vi "CRYO_MASTER_FULL_dev.vi"() -> ()   [LabVIEW 2017] (continued)
  out "P (1K pot)":dbl=100068.27348256127 format="%_4e"
  out "P (3He pot)":dbl=99910.45562672244 format="%_4e"
  out "P (shield return)":dbl=99525.03881922836 format="%_4e"
  out "P (3He IN)":dbl=99868.7240011457 format="%_4e"
  out "P (4K reservoir)":dbl=99802.94678056413 format="%_4e"
  out "P (insulation)":dbl=0.0001474505418094343 format="%_4e"
  in  "1Kpot pump exhaust flow":string="F_5"
  out "F_5":dbl=37.619829557129414 format="%_4f"
  in  "3He incoming flow into HEX7":string="F_4"
  out "F_4":dbl=-7.249983269540847 format="%_4f"
  out "F_3":dbl=-0.052681534547558584 format="%_4f"
  in  "4He return flow from HEX7":string="F_3"
  out "F_2":dbl=-0.13159086515246687 format="%_4f"
  in  "Shield flow":string="F_2"
  out "P_SldRTN":dbl=99525.03881922836 format="%_4e"
  in  "3He pot pressure":string="P_3Hepot"
  out "P_3Hepot":dbl=99910.45562672244 format="%_4e"
  in  "Shield return press.":string="P_SldRTN"
  out "F_1":dbl=3.609913543945148 format="%_4f"
  in  "3He pump exhaust flow":string="F_1"
  out "P_Dewar":dbl=100437.10701708468 format="%_4e"
  in  "Dewar pressure":string="P_Dewar"
  out "P_1Kpot":dbl=100068.27348256127 format="%_4e"
  in  "1Kpot pressure":string="P_1Kpot"
  out "P_3HeIN":dbl=99868.7240011457 format="%_4e"
  in  "3He inlet pressure":string="P_3HeIN"
  in  "4K reservoir pressure":string="P_4Kres"
  out "P_4Kres":dbl=99802.94678056413 format="%_4e"
  out "P_ins":dbl=0.0001474505418094343 format="%_4e"
  in  "Insulation vacuum":string="P_ins"
  out "T3He7-1/6-2 (3He pot) 2":dbl=8.3718 format="%_4f"
  out "T3He7-1/7-2 (HEX1)":dbl=8.4614 format="%_4f"
  out "T3He6-1/6-2 (3He pot) 2":dbl=8.4997 format="%_4f"
  out "T3He6-1/6-2 (HEX1)":dbl=8.4934 format="%_4f"
  out "T1K3-1/3-2 (1K pot) 2":dbl=4.1883 format="%_4f"
  out "T1K3-1/3-2 (1K pot)":dbl=4.1814 format="%_4f"
  out "T4He1 (4K reservoir )":dbl=4.447 format="%_4f"
  out "Temperature 1":dbl=19.065
  in  "SensorLocation 1":T14(ring)=enum."TTH2"
  out "TIP7":dbl format="%_4g"
  out "T3He6-2":dbl=8.4997 format="%_4g"
  out "T3He7-2":dbl=8.3718 format="%_4g"
  out "T3He6-1":dbl=8.4934 format="%_4g"
  out "T3He4":dbl=9.675 format="%_4g"
  out "T3He7-1":dbl=8.4614 format="%_4g"
  out "T3He8":dbl=8.8291 format="%_4g"
  out "T3He5":dbl=4.3215 format="%_4g"
  out "T1K3-2":dbl=4.1883 format="%_4g"
  out "T1K3-1":dbl=4.1814 format="%_4g"
  out "TIP6":dbl=18.257 format="%_4g"
  out "T3He9":dbl=10.682 format="%_4g"
  out "T1K5":dbl=4.692 format="%_4g"
  out "T1K4":dbl=4.458 format="%_4g"
  out "T1K2":dbl=4.216 format="%_4g"
  out "TIP5":dbl=17.346 format="%_4g"
  out "TIP4":dbl=11.053 format="%_4g"
  out "TIP3":dbl=39.061 format="%_4g"
  out "TIP2":dbl=88.205 format="%_4g"
  out "TIP1":dbl=246.21 format="%_4g"
  out "T1K6":dbl=250.44 format="%_4g"
  out "T4He10":dbl=208.38 format="%_4g"
  out "T4He8":dbl=166.06 format="%_4g"
  out "T4He7":dbl=115.68 format="%_4g"
  out "T3He1-3":dbl=277.53 format="%_4g"
  out "T3He1-2":dbl=279.51 format="%_4g"
  out "T4He9":dbl=97.885 format="%_4g"
  out "T4He6":dbl=25.122 format="%_4g"
  out "T4He5":dbl=25.726 format="%_4g"
  out "T4He4":dbl=30.925 format="%_4g"
  out "T4He2-2":dbl=35.069 format="%_4g"
  out "T4He2-1":dbl=34.286 format="%_4g"
  out "T4He3-4":dbl=285.55 format="%_4g"
  out "T4He3-3":dbl=285.5 format="%_4g"
  out "T4He3-2":dbl=287.85 format="%_4g"
  out "T4He3-1":dbl=287.74 format="%_4g"
  out "T3He1-4":dbl=276.97 format="%_4g"
  out "T3He3":dbl=17.248 format="%_4g"
  out "T3He2-2":dbl=34.793 format="%_4g"
  out "T3He2-1":dbl=46.023 format="%_4g"
  out "T1K1":dbl=10.801 format="%_4g"
  out "T4He1":dbl=4.447 format="%_4g"
  out "TTH1":dbl=19.184 format="%_4g"
  out "TTH2":dbl=19.065 format="%_4g"
  out "TTH4":dbl=112.53 format="%_4g"
  out "TTH3":dbl=106.31 format="%_4g"
  out "T3He1-1":dbl=279.64 format="%_4g"
  out "T3He10":dbl=250.64 format="%_4g"
  out "F2 (shield flow)":dbl=-0.13159086515246687 format="%_4f"
  out "DP_HEX4":dbl=-42.27649010016066 format="%_4e"
  in  "4K reservoir level":string="L3"
  out "L3":dbl=0.05537433565456876 format="%_4f"
  out "RUN Identifier 6":string="20201120_195613_RUNII" caption="RUN Identifier"
  in  "HEX7 out pressure":string="P_HEX7OUT"
  in  "STOP CHF":bool
  in  "CHF Graph Comment":string="CHF_Warmup"
  in  "REFRESH GRAPH":bool
  in  "RECORD GRAPH":bool
  out "Graph CHF log 2":T4(graph) caption="XY Graph"
  out "ƒ¢T_array":dbl[](array[numeric])=[-0.0029999999999998916, -0.0031999999999998696, -0.0031999999999998696, -0.0031999999999998696, -0.0030999999999998806, -0.0030999999999998806, -0.0031999999999998696, -0.0033999999999998476, -0.0030999999999998806, -0.0032999999999998586, -0.0028999999999999027, -0.0032999999999998586, -0.0030999999999998806, -0.0032999999999998586, -0.0030999999999998806, -0.0030999999999998806, -0.0030999999999998806, -0.0031999999999998696, -0.0031999999999998696, -0.0029999999999998916, -0.0028999999999999027, -0.0029999999999998916, -0.0032000000000000917, -0.0030000000000001137, -0.0031000000000001027, -0.0027000000000001467, -0.0029000000000001247, -0.0029000000000001247, -0.0031000000000001027, -0.0025999999999999357, -0.0027999999999999137, -0.0025999999999999357, -0.0027999999999999137, -0.0024999999999999467, -0.0028999999999999027, -0.0023999999999999577, -0.0023000000000001908, -0.0023999999999999577, -0.0026999999999999247, -0.0024999999999999467, -0.0023999999999999577, -0.0024999999999999467, -0.0023999999999999577, -0.0025000000000001688, -0.0020000000000000018, -0.0022999999999999687, -0.002100000000000213, -0.0020000000000000018, -0.0020999999999999908, -0.0016000000000000458, -0.0019000000000000128, -0.0014000000000000679, -0.0017000000000000348, -0.0013000000000000789, -0.0013999999999998458, -0.0011999999999998678, -0.0016000000000000458, -0.0017000000000000348, -0.0009000000000001229, -0.0012000000000000899, -0.0008000000000001339, -0.001000000000000112, -0.0012000000000000899, -0.0010999999999998789, -0.0009000000000001229, -0.0010999999999998789, -0.0019000000000000128, -0.0016000000000000458, -0.0008999999999999009, -0.0004999999999999449, -0.0009000000000001229, -0.0011999999999998678, -0.0006999999999997009, -0.00010000000000021103, -0.0010999999999996568, -0.001100000000000101, -0.0008999999999996788, 0.00010000000000021103, -0.000700000000000145, -0.00039999999999995595, 0.0, -0.00010000000000021103, 0.00019999999999997797, -0.0009999999999998899, 0.00019999999999997797, -0.000700000000000145, 0.000600000000000378, -0.0006999999999997009, 0.0015999999999998238, 0.0015999999999998238, 0.010199999999999765, 0.00140000000000029, 0.0038999999999997925, -0.007899999999999796, 0.0028999999999999027, -0.004100000000000215, 0.006000000000000227, 0.0034000000000000696, 0.0, -0.0026000000000001577, 0.0013000000000000789, -0.013700000000000045, 0.0015000000000000568, 0.0038000000000000256, 0.000300000000000189, -0.0034000000000000696, -0.00019999999999997797, -0.0009000000000001229, -0.0049000000000001265, -0.0017000000000000348, 0.0020999999999999908, 0.000700000000000145, 0.0024999999999999467, 0.0011999999999998678, 0.0043999999999999595, 0.001200000000000312, -0.0009999999999998899, -0.00039999999999995595, 0.0027999999999996916, 0.0020999999999999908, 0.0028000000000001357, 0.0028000000000001357, 0.0038000000000000256, 0.006200000000000205, 0.001100000000000101, 0.0040000000000000036, 0.0024999999999999467, 0.005300000000000082, 0.0027000000000003688, 0.0032000000000000917, 0.0046000000000003816, 0.0045000000000001705, 0.00550000000000006, 0.0038999999999997925, 0.0045999999999999375, 0.0032999999999998586, 0.0039000000000002366, 0.0028000000000001357, 0.0019999999999997797, 0.0040000000000000036, 0.0013999999999998458, 0.006600000000000161, 0.0015999999999998238, 0.0045000000000001705, 0.02400000000000002, 0.012199999999999989, 0.0049000000000001265, 0.014599999999999724, 0.0043999999999999595, 0.013900000000000023, 0.007899999999999796, 0.014200000000000212, 0.08460000000000001, 0.0038000000000000256, 0.014199999999999768, 0.029699999999999616, 0.051200000000000134, 0.09330000000000016, 0.28469999999999995, 1.3064, 0.7519, 0.9085000000000001, 3.6559, 3.1087999999999996, 3.1484000000000005, 4.376900000000001, 4.8179, 5.180999999999999, 5.6812000000000005, 6.102599999999999, 6.5953, 6.675800000000001, 7.3666, 7.8156, 8.344, 8.904599999999999, 8.9488, 9.2997, 9.7916, 10.0504, 10.446399999999999, 10.966099999999999, 11.3154, 11.6655, 12.011, 12.4506, 12.629000000000001, 12.9298, 13.34, 13.658900000000001, 14.0009, 14.365399999999998, 14.6644, 14.959400000000002, 15.242600000000001, 15.613299999999999, 15.9224, 16.2284, 16.4516, 16.7094]
  out "Graph CHF":cluster{dbl[], dbl[]}(graph)={[-0.0029999999999998916, -0.0031999999999998696, -0.0031999999999998696, -0.0031999999999998696, -0.0030999999999998806, -0.0030999999999998806, -0.0031999999999998696, -0.0033999999999998476, -0.0030999999999998806, -0.0032999999999998586, -0.0028999999999999027, -0.0032999999999998586, -0.0030999999999998806, -0.0032999999999998586, -0.0030999999999998806, -0.0030999999999998806, -0.0030999999999998806, -0.0031999999999998696, -0.0031999999999998696, -0.0029999999999998916, -0.0028999999999999027, -0.0029999999999998916, -0.0032000000000000917, -0.0030000000000001137, -0.0031000000000001027, -0.0027000000000001467, -0.0029000000000001247, -0.0029000000000001247, -0.0031000000000001027, -0.0025999999999999357, -0.0027999999999999137, -0.0025999999999999357, -0.0027999999999999137, -0.0024999999999999467, -0.0028999999999999027, -0.0023999999999999577, -0.0023000000000001908, -0.0023999999999999577, -0.0026999999999999247, -0.0024999999999999467, -0.0023999999999999577, -0.0024999999999999467, -0.0023999999999999577, -0.0025000000000001688, -0.0020000000000000018, -0.0022999999999999687, -0.002100000000000213, -0.0020000000000000018, -0.0020999999999999908, -0.0016000000000000458, -0.0019000000000000128, -0.0014000000000000679, -0.0017000000000000348, -0.0013000000000000789, -0.0013999999999998458, -0.0011999999999998678, -0.0016000000000000458, -0.0017000000000000348, -0.0009000000000001229, -0.0012000000000000899, -0.0008000000000001339, -0.001000000000000112, -0.0012000000000000899, -0.0010999999999998789, -0.0009000000000001229, -0.0010999999999998789, -0.0019000000000000128, -0.0016000000000000458, -0.0008999999999999009, -0.0004999999999999449, -0.0009000000000001229, -0.0011999999999998678, -0.0006999999999997009, -0.00010000000000021103, -0.0010999999999996568, -0.001100000000000101, -0.0008999999999996788, 0.00010000000000021103, -0.000700000000000145, -0.00039999999999995595, 0.0, -0.00010000000000021103, 0.00019999999999997797, -0.0009999999999998899, 0.00019999999999997797, -0.000700000000000145, 0.000600000000000378, -0.0006999999999997009, 0.0015999999999998238, 0.0015999999999998238, 0.010199999999999765, 0.00140000000000029, 0.0038999999999997925, -0.007899999999999796, 0.0028999999999999027, -0.004100000000000215, 0.006000000000000227, 0.0034000000000000696, 0.0, -0.0026000000000001577, 0.0013000000000000789, -0.013700000000000045, 0.0015000000000000568, 0.0038000000000000256, 0.000300000000000189, -0.0034000000000000696, -0.00019999999999997797, -0.0009000000000001229, -0.0049000000000001265, -0.0017000000000000348, 0.0020999999999999908, 0.000700000000000145, 0.0024999999999999467, 0.0011999999999998678, 0.0043999999999999595, 0.001200000000000312, -0.0009999999999998899, -0.00039999999999995595, 0.0027999999999996916, 0.0020999999999999908, 0.0028000000000001357, 0.0028000000000001357, 0.0038000000000000256, 0.006200000000000205, 0.001100000000000101, 0.0040000000000000036, 0.0024999999999999467, 0.005300000000000082, 0.0027000000000003688, 0.0032000000000000917, 0.0046000000000003816, 0.0045000000000001705, 0.00550000000000006, 0.0038999999999997925, 0.0045999999999999375, 0.0032999999999998586, 0.0039000000000002366, 0.0028000000000001357, 0.0019999999999997797, 0.0040000000000000036, 0.0013999999999998458, 0.006600000000000161, 0.0015999999999998238, 0.0045000000000001705, 0.02400000000000002, 0.012199999999999989, 0.0049000000000001265, 0.014599999999999724, 0.0043999999999999595, 0.013900000000000023, 0.007899999999999796, 0.014200000000000212, 0.08460000000000001, 0.0038000000000000256, 0.014199999999999768, 0.029699999999999616, 0.051200000000000134, 0.09330000000000016, 0.28469999999999995, 1.3064, 0.7519, 0.9085000000000001, 3.6559, 3.1087999999999996, 3.1484000000000005, 4.376900000000001, 4.8179, 5.180999999999999, 5.6812000000000005, 6.102599999999999, 6.5953, 6.675800000000001, 7.3666, 7.8156, 8.344, 8.904599999999999, 8.9488, 9.2997, 9.7916, 10.0504, 10.446399999999999, 10.966099999999999, 11.3154, 11.6655, 12.011, 12.4506, 12.629000000000001, 12.9298, 13.34, 13.658900000000001, 14.0009, 14.365399999999998, 14.6644, 14.959400000000002, 15.242600000000001, 15.613299999999999, 15.9224, 16.2284, 16.4516, 16.7094], [0.00177179408, 0.0047188563824, 0.009062122761600002, 0.014841429971200002, 0.022050593188799993, 0.030674497986, 0.0406770254784, 0.0520756828592, 0.0652426793424, 0.07951245148399999, 0.095196614256, 0.11212304208000001, 0.13146225656, 0.15140636999200002, 0.172767285228, 0.19523839632000003, 0.22089373680000002, 0.24639792231999996, 0.27309037243199996, 0.300834606864, 0.333309042144, 0.364200416856, 0.396376777992, 0.428969786608, 0.46852352470399994, 0.5048892, 0.5415947771520001, 0.5780588070400001, 0.62555439864, 0.6656076272399999, 0.7053064507, 0.7438503797200001, 0.8028658319759999, 0.84516135816, 0.8855220791599998, 0.9243742466799998, 0.9987769028, 1.040549527104, 1.07657183264, 1.1053520089920001, 1.2023590229040002, 1.3125317079600003, 1.355469355336, 1.4108726480399998, 1.4642265462839996, 1.5508259575799999, 1.609969226688, 1.6681944120439995, 1.7212315581999997, 1.8197203732960001, 1.8816147001599999, 1.939246332968, 1.993681569632, 2.110421822528, 2.1715208164760003, 2.2300658826359996, 2.33203464608, 2.4312324865440003, 2.520524222848, 2.56333261656, 2.661313337984, 2.7867724064, 2.8377456422800003, 2.963749773600001, 3.01323235824, 3.143606416840001, 3.1874947393199995, 3.3286276941600006, 3.3671324332799997, 3.4297475918799996, 3.4776642959999995, 3.48994194976, 3.7174310035199993, 3.7518448211999993, 3.756501273839999, 3.8155461344, 4.26509900712, 4.04162726208, 4.09879309824, 4.5867353948, 4.69579370944, 4.39389811152, 4.9172907186399994, 5.029857857199999, 5.14319635, 5.257784033319999, 5.373066988079999, 5.48922905748, 5.606999167360001, 5.7253151114400005, 5.8451341704, 5.9653806828, 6.087172249440001, 6.20936272008, 6.3330874655999985, 6.457355812319998, 6.5829079103599994, 6.709043396000002, 6.836579179000002, 6.9645565727999985, 7.093596729600001, 7.223932919599999, 7.354796004800001, 7.486911963999998, 7.6198231199999995, 7.7532066848, 7.887716202000003, 8.024043540800001, 8.126487840000001, 8.269554521199998, 8.4077936336, 8.5471331664, 8.6875860064, 8.8284394528, 8.971763136, 9.114345182800001, 9.257739612, 9.403949720000002, 9.549304752000001, 9.695266022, 9.841513750000003, 9.99153291, 10.140170450400001, 10.289093019200001, 10.4378083004, 10.594207987199999, 10.7454584848, 10.897314274, 11.0478970848, 11.210433023999999, 11.363073264000002, 11.514230988000001, 11.6672069304, 11.8363924328, 11.990053261999998, 12.141437804, 12.316577644799997, 12.469949637600003, 12.6221502, 12.768815616000001, 12.9613889756, 13.112679096, 13.260713388, 13.3955342568, 13.6139294592, 13.767960665600002, 13.903996679999999, 14.0298325128, 14.272124848799997, 14.408208115599999, 14.535468526799997, 14.625996168000002, 14.9276629944, 15.049154579999998, 15.132236211999997, 15.444088045600003, 15.570016308800001, 15.687675859999997, 15.778474975199998, 16.133452762, 16.2316771404, 16.278357173599996, 16.259788331199996, 16.7384176632, 16.723491475199996, 16.714044836000003, 16.528176336, 17.254680908799997, 18.0156484144, 16.952834118, 18.4038018464, 18.599578232000002, 18.794163826000002, 18.99096738, 19.1888872744, 19.3889457516, 19.588486306799997, 19.789104642, 19.9907612412, 20.1933504, 20.396427222400003, 20.600519206399998, 20.8041637608, 21.010700178, 21.216750239999996, 21.4245511792, 21.632564418399998, 21.8418047652, 22.051294878, 22.26281235, 22.47403692, 22.68618526, 22.899439349999998, 23.111589312, 23.325939447999996, 23.540653440000003, 23.7536142072, 23.968794931199998, 24.183715353199997, 24.407023065599997]}
  in  "V_lim_low (V)":dbl format="%_5f"
  in  "V_lim_up (V)":dbl=120.0 format="%_5f"
  out "V":dbl=37.9024
  out "I":dbl=0.643944
  out "Q":dbl=24.407023065599997
  out "T_low":dbl=2.1656
  out "CHF log file name":string="20201120_102906_RUNII_20201120_154856_CHFlog.csv"
  in  "Data T_low":T15={"Source"=enum."LSI336", "SourceLabel"="T3He6-1"}
  in  "Data T_high":T15={"Source"=enum."LSI336", "SourceLabel"="T3He7-2"}
  in  "RecordSettings":T16(array[cluster])=[{"Source"=enum."DMMs", "SourceLabel"="I_H1", "FileFormat"="%4.4e"}, {"Source"=enum."DMMs", "SourceLabel"="V_H1", "FileFormat"="%4.4f"}, {"Source"=enum."USB6210", "SourceLabel"="P_3Hepot", "FileFormat"="%4.4e"}, {"Source"=enum."USB6218AI", "SourceLabel"="F_1", "FileFormat"="%4.4f"}, {"Source"=enum."USB6218AI", "SourceLabel"="F_4", "FileFormat"="%4.4f"}, {"Source"=enum."USB6218AI", "SourceLabel"="F_5", "FileFormat"="%4.4f"}, {"Source"=enum."USB6210", "SourceLabel"="DP_HEX4", "FileFormat"="%4.4e"}, {"Source"=enum."LSI336", "SourceLabel"="T3He6-1", "FileFormat"="%4.4f"}, {"Source"=enum."LSI336", "SourceLabel"="T3He6-2", "FileFormat"="%4.4f"}, {"Source"=enum."LSI336", "SourceLabel"="T3He7-1", "FileFormat"="%4.4f"}, {"Source"=enum."LSI336", "SourceLabel"="T3He7-2", "FileFormat"="%4.4f"}, {"Source"=enum."LSI336", "SourceLabel"="T1K3-1", "FileFormat"="%4.4f"}, {"Source"=enum."LSI336", "SourceLabel"="T1K3-2", "FileFormat"="%4.4f"}]
  in  "Data V":T15={"Source"=enum."DMMs", "SourceLabel"="V_H1"}
  in  "Data I":T15={"Source"=enum."DMMs", "SourceLabel"="I_H1"}
  in  "START CHF":bool
  in  "CHF cycle interval (s) (>1s)":dbl=1.0 format="%_3f"
  in  "V_end (V)":dbl=100.0 format="%_4f"
  in  "V start (V)":dbl format="%_4f"
  in  "ƒ¢V / cycle (V)":dbl=0.5 format="%_4f"
  out "error out (Agilent)":errorcluster
  in  "VISA (Agilent 34402)":refnum<visa-resource-name>="USB0::0x0957::0x0407::MY44010230::INSTR"
  out "Agilent\nIntialized?":bool=TRUE
  in  "Initialize (Agilent)":bool
  in  "OUTPUT \nKenwood":bool
  in  "Kenwood set V (V)":dbl min=0.0 max=120.0 format="%_5f"
  out "Graph CHF log 1":T4(graph) caption="XY Graph"
  out "CHF Data Labels":string[](array[string])=["I_H1", "V_H1", "P_3Hepot", "F_1", "F_4", "F_5", "DP_HEX4", "T3He6-1", "T3He6-2", "T3He7-1", "T3He7-2", "T1K3-1", "T1K3-2"]
  out "CHF last data":dbl[](array[numeric])=[0.643944, 37.9024, 3745.6366507925286, 1.653619757825851, -6.92448226263659, 35.2098077546946, -11.781018947359195, 2.1656, 6.7476, 2.1606, 18.875, 1.9567, 1.9598]
  out "Error out (CHF rec)":errorcluster
  out "CHF measurement counter":i32
  out "T_high":dbl=18.875
  out "ƒ¢T":dbl=16.7094
  out "Q_array":dbl[](array[numeric])=[0.00177179408, 0.0047188563824, 0.009062122761600002, 0.014841429971200002, 0.022050593188799993, 0.030674497986, 0.0406770254784, 0.0520756828592, 0.0652426793424, 0.07951245148399999, 0.095196614256, 0.11212304208000001, 0.13146225656, 0.15140636999200002, 0.172767285228, 0.19523839632000003, 0.22089373680000002, 0.24639792231999996, 0.27309037243199996, 0.300834606864, 0.333309042144, 0.364200416856, 0.396376777992, 0.428969786608, 0.46852352470399994, 0.5048892, 0.5415947771520001, 0.5780588070400001, 0.62555439864, 0.6656076272399999, 0.7053064507, 0.7438503797200001, 0.8028658319759999, 0.84516135816, 0.8855220791599998, 0.9243742466799998, 0.9987769028, 1.040549527104, 1.07657183264, 1.1053520089920001, 1.2023590229040002, 1.3125317079600003, 1.355469355336, 1.4108726480399998, 1.4642265462839996, 1.5508259575799999, 1.609969226688, 1.6681944120439995, 1.7212315581999997, 1.8197203732960001, 1.8816147001599999, 1.939246332968, 1.993681569632, 2.110421822528, 2.1715208164760003, 2.2300658826359996, 2.33203464608, 2.4312324865440003, 2.520524222848, 2.56333261656, 2.661313337984, 2.7867724064, 2.8377456422800003, 2.963749773600001, 3.01323235824, 3.143606416840001, 3.1874947393199995, 3.3286276941600006, 3.3671324332799997, 3.4297475918799996, 3.4776642959999995, 3.48994194976, 3.7174310035199993, 3.7518448211999993, 3.756501273839999, 3.8155461344, 4.26509900712, 4.04162726208, 4.09879309824, 4.5867353948, 4.69579370944, 4.39389811152, 4.9172907186399994, 5.029857857199999, 5.14319635, 5.257784033319999, 5.373066988079999, 5.48922905748, 5.606999167360001, 5.7253151114400005, 5.8451341704, 5.9653806828, 6.087172249440001, 6.20936272008, 6.3330874655999985, 6.457355812319998, 6.5829079103599994, 6.709043396000002, 6.836579179000002, 6.9645565727999985, 7.093596729600001, 7.223932919599999, 7.354796004800001, 7.486911963999998, 7.6198231199999995, 7.7532066848, 7.887716202000003, 8.024043540800001, 8.126487840000001, 8.269554521199998, 8.4077936336, 8.5471331664, 8.6875860064, 8.8284394528, 8.971763136, 9.114345182800001, 9.257739612, 9.403949720000002, 9.549304752000001, 9.695266022, 9.841513750000003, 9.99153291, 10.140170450400001, 10.289093019200001, 10.4378083004, 10.594207987199999, 10.7454584848, 10.897314274, 11.0478970848, 11.210433023999999, 11.363073264000002, 11.514230988000001, 11.6672069304, 11.8363924328, 11.990053261999998, 12.141437804, 12.316577644799997, 12.469949637600003, 12.6221502, 12.768815616000001, 12.9613889756, 13.112679096, 13.260713388, 13.3955342568, 13.6139294592, 13.767960665600002, 13.903996679999999, 14.0298325128, 14.272124848799997, 14.408208115599999, 14.535468526799997, 14.625996168000002, 14.9276629944, 15.049154579999998, 15.132236211999997, 15.444088045600003, 15.570016308800001, 15.687675859999997, 15.778474975199998, 16.133452762, 16.2316771404, 16.278357173599996, 16.259788331199996, 16.7384176632, 16.723491475199996, 16.714044836000003, 16.528176336, 17.254680908799997, 18.0156484144, 16.952834118, 18.4038018464, 18.599578232000002, 18.794163826000002, 18.99096738, 19.1888872744, 19.3889457516, 19.588486306799997, 19.789104642, 19.9907612412, 20.1933504, 20.396427222400003, 20.600519206399998, 20.8041637608, 21.010700178, 21.216750239999996, 21.4245511792, 21.632564418399998, 21.8418047652, 22.051294878, 22.26281235, 22.47403692, 22.68618526, 22.899439349999998, 23.111589312, 23.325939447999996, 23.540653440000003, 23.7536142072, 23.968794931199998, 24.183715353199997, 24.407023065599997]
  out "CHF file name":string="20201120_102906_RUNII_CHF20201120_155319_CHF_Warmup.csv"
  out "Graph CHF log 3":T4(graph) caption="XY Graph"
  out "File Refnum (CHF)":refnum<file>
  out "Series 1":string[](array[string])=["P_ins", "P_4Kres", "P_3HeIN", "P_SldRTN", "P_3Hepot", "P_1Kpot", "P_Dewar(old)", "P_HEX7OUT", "P_IP"]
  out "Series 2":string[](array[string])=["DP_HEX4", "DP_HEX5", "L1", "L2-1", "L2-2", "L3"]
  out "Series 3":string[](array[string])=["F_1", "F_2", "F_3", "F_4", "F_5", "I_CV", "P_Dewar"]
  out "Series 4":string[](array[string])=["TTH3", "TTH4", "TTH1", "TTH2", "T4He1", "T1K1", "T3He2-1", "T3He2-2", "T4He3-1", "T4He3-2", "T4He3-3", "T4He3-4", "T4He2-1", "T4He2-2", "T4He4", "T1K2", "T1K4", "T1K5", "T3He4", "T1K3-1", "T1K3-2", "T3He5", "T3He8", "T3He6-1", "T3He6-2", "T3He7-1", "T3He7-2"]
  out "Plot errors":errorcluster
  out "LastMeasurementConfig (218)":T17(array[cluster])=[{"LSIName"="LSI218A", "Active?"=TRUE, "LastData"=[250.64, 279.64, 106.3, 112.52, 19.165, 19.038, 4.436, 10.775], "Labels"=["T3He10", "T3He1-1", "TTH3", "TTH4", "TTH1", "TTH2", "T4He1", "T1K1"]}, {"LSIName"="LSI218B", "Active?"=TRUE, "LastData"=[30.0, 0.0, 0.0, 0.0, 46.025, 34.792, 17.25, 276.96], "Labels"=["N.C.", "N.C.", "N.C.", "N.C.", "T3He2-1", "T3He2-2", "T3He3", "T3He1-4"]}, {"LSIName"="LSI218C", "Active?"=TRUE, "LastData"=[287.74, 287.84, 285.5, 285.55, 34.292, 35.074, 30.928, 25.728], "Labels"=["T4He3-1", "T4He3-2", "T4He3-3", "T4He3-4", "T4He2-1", "T4He2-2", "T4He4", "T4He5"]}, {"LSIName"="LSI218D", "Active?"=TRUE, "LastData"=[25.125, 97.886, 279.52, 277.53, 115.69, 166.07, 208.39, 250.44], "Labels"=["T4He6", "T4He9", "T3He1-2", "T3He1-3", "T4He7", "T4He8", "T4He10", "T1K6"]}, {"LSIName"="LSI218E", "Active?"=TRUE, "LastData"=[246.21, 0.0, 88.2, 688.49, 39.062, 11.046, 17.368, 688.58], "Labels"=["TIP1", "N.C.", "TIP2", "N.C.", "TIP3", "TIP4", "TIP5", "N.C."]}, {"LSIName"="LSI218F", "Active?"=TRUE, "LastData"=[4.194, 4.476, 4.691, 9.636, 10.639, 18.262, 0.433, 0.0], "Labels"=["T1K2", "T1K4", "T1K5", "T3He4", "T3He9", "TIP6", "N.C.", "N.C."]}]
  out "DataArrayConv (USB6210)":dbl[][](array[numeric])
  out "LastMeasurementConfig (336)":T17(array[cluster])=[{"LSIName"="LSi336X", "Active?"=TRUE, "LastData"=[4.182, 4.1886, 4.3213, 8.8312], "Labels"=["T1K3-1", "T1K3-2", "T3He5", "T3He8"]}, {"LSIName"="LSi336Y", "Active?"=TRUE, "LastData"=[8.4926, 8.5004, 8.4614, 8.3712], "Labels"=["T3He6-1", "T3He6-2", "T3He7-1", "T3He7-2"]}]
  out "DataArrayConv (USB6218)":dbl[][](array[numeric])
  out "TimeArray (USB6218)":timestamp[](array[timestamp])
  out "Data Array sizes (6210)":i32[](array[numeric])=[33552, 16]
  out "DataArraySize (6218)":i32[](array[numeric])=[33552, 8]
  out "TimeArray size (6218)":i32=33552
  out "TimeArray (LSI336)":timestamp[](array[timestamp])
  out "TimeArray Size (336)":i32=33552
  out "DataArray (336)":dbl[][](array[numeric])
  out "DataArray size (336)":i32[](array[numeric])=[33552, 8]
  out "LastData (LSI218)":dbl[](array[numeric])=[250.64, 279.64, 106.3, 112.52, 19.165, 19.038, 4.436, 10.775, 30.0, 0.0, 0.0, 0.0, 46.025, 34.792, 17.25, 276.96, 287.74, 287.84, 285.5, 285.55, 34.292, 35.074, 30.928, 25.728, 25.125, 97.886, 279.52, 277.53, 115.69, 166.07, 208.39, 250.44, 246.21, 0.0, 88.2, 688.49, 39.062, 11.046, 17.368, 688.58, 4.194, 4.476, 4.691, 9.636, 10.639, 18.262, 0.433, 0.0]
  out "TempSensorsLocations":T18(array[ring])=[enum."T3He10", enum."T3He1-1", enum."TTH3", enum."TTH4", enum."TTH1", enum."TTH2", enum."T4He1", enum."T1K1", enum."N.C.", enum."N.C.", enum."N.C.", enum."N.C.", enum."T3He2-1", enum."T3He2-2", enum."T3He3", enum."T3He1-4", enum."T4He3-1", enum."T4He3-2", enum."T4He3-3", enum."T4He3-4", enum."T4He2-1", enum."T4He2-2", enum."T4He4", enum."T4He5", enum."T4He6", enum."T4He9", enum."T3He1-2", enum."T3He1-3", enum."T4He7", enum."T4He8", enum."T4He10", enum."T1K6", enum."TIP1", enum."N.C.", enum."TIP2", enum."N.C.", enum."TIP3", enum."TIP4", enum."TIP5", enum."N.C.", enum."T1K2", enum."T1K4", enum."T1K5", enum."T3He4", enum."T3He9", enum."TIP6", enum."N.C.", enum."N.C.", enum."T1K3-1", enum."T1K3-2", enum."T3He5", enum."T3He8", enum."T3He6-1", enum."T3He6-2", enum."T3He7-1", enum."T3He7-2"]
  out "AllTemperatures":dbl[](array[numeric])=[250.64, 279.64, 106.31, 112.53, 19.184, 19.065, 4.447, 10.801, 30.0, 0.0, 0.0, 0.0, 46.023, 34.793, 17.248, 276.97, 287.74, 287.85, 285.5, 285.55, 34.286, 35.069, 30.925, 25.726, 25.122, 97.885, 279.51, 277.53, 115.68, 166.06, 208.38, 250.44, 246.21, 0.0, 88.205, 688.49, 39.061, 11.053, 17.346, 688.58, 4.216, 4.458, 4.692, 9.675, 10.682, 18.257, 0.433, 0.0, 4.1814, 4.1883, 4.3215, 8.8291, 8.4934, 8.4997, 8.4614, 8.3718]
  out "error out (frontpanel screenshots)":errorcluster
  out "error out (graph operations)":errorcluster
  out "error out (monthly folder creation)":errorcluster={"status"=TRUE, "code"=10, "source"="Create Folder in CRYO_MASTER_FULL_dev.vi<APPEND>\nC:\\LabVIEW\\DATA\\Google\\TUCAN Experiments\\KEK_cryotests_2019-2020\\data\\screenshots\\202011"}
  out "RUN Identifier 7":string="20201120_195613_RUNII" caption="RUN Identifier"
  out "error out (notifier)":errorcluster
  # "GLOBAL STATUS/CONTROL"
  # "Global Settings"
  # "USB6210 Analog inputs Settings"
  # "USB6218 Analog inputs Settings"
  # "USB6218 Digital Output Settings"
  # "USB6218 Analog Output Settings"
  # "LSI218 Settings"
  # "LSI336 Settings"
  # "HP 34401A (He level meter)"
  # "Graph screenshots"
  # "Configuration"
  # "Activated only when *FIll state* = TRUE"
  # "Activated only when *FIll state* = TRUE"
  # "Vavle Status"
  # "OPEN"
  # "CLOSED"
  # "ADCMT6240A Control/Status"
  # "ADCMT6240A Initialization"
  # "Set Currents (mA)"
  # "PWR400H CTRL via USB6218"
  # "PMC18-3A CTRL via USB621"
  # "DMM configurations"
  # "DMM measurements"
  # "CAUTION: ADCMT 7351 does not have 4-wire resistance measurement function. \n 4-Wire Resistance --> 2-Wire Resistance wih Low Power for this device"
  # "Representative temperatures"
  # "Pressures / Flows"
  # "Labels"
  # "Values"
  # "Helium Levels"
  # "Manual Control of Kenwood"
  # "Automatic Measurement"
  # "Before the measurement\n - Intialize Agilent 34402 (FG)\n - Refresh the CHF graph if necessary\n - Go to DMMs tab and check that DMM measurement is running \n - Fill in the CHF measurement parameters below \nThen press START CHF!"
  # "Measurement Configurations"
  # "Channel selection"
  # "Q = I x V"
  # "ƒ¢T = T_high - T_low"
  # "Record Configurations"
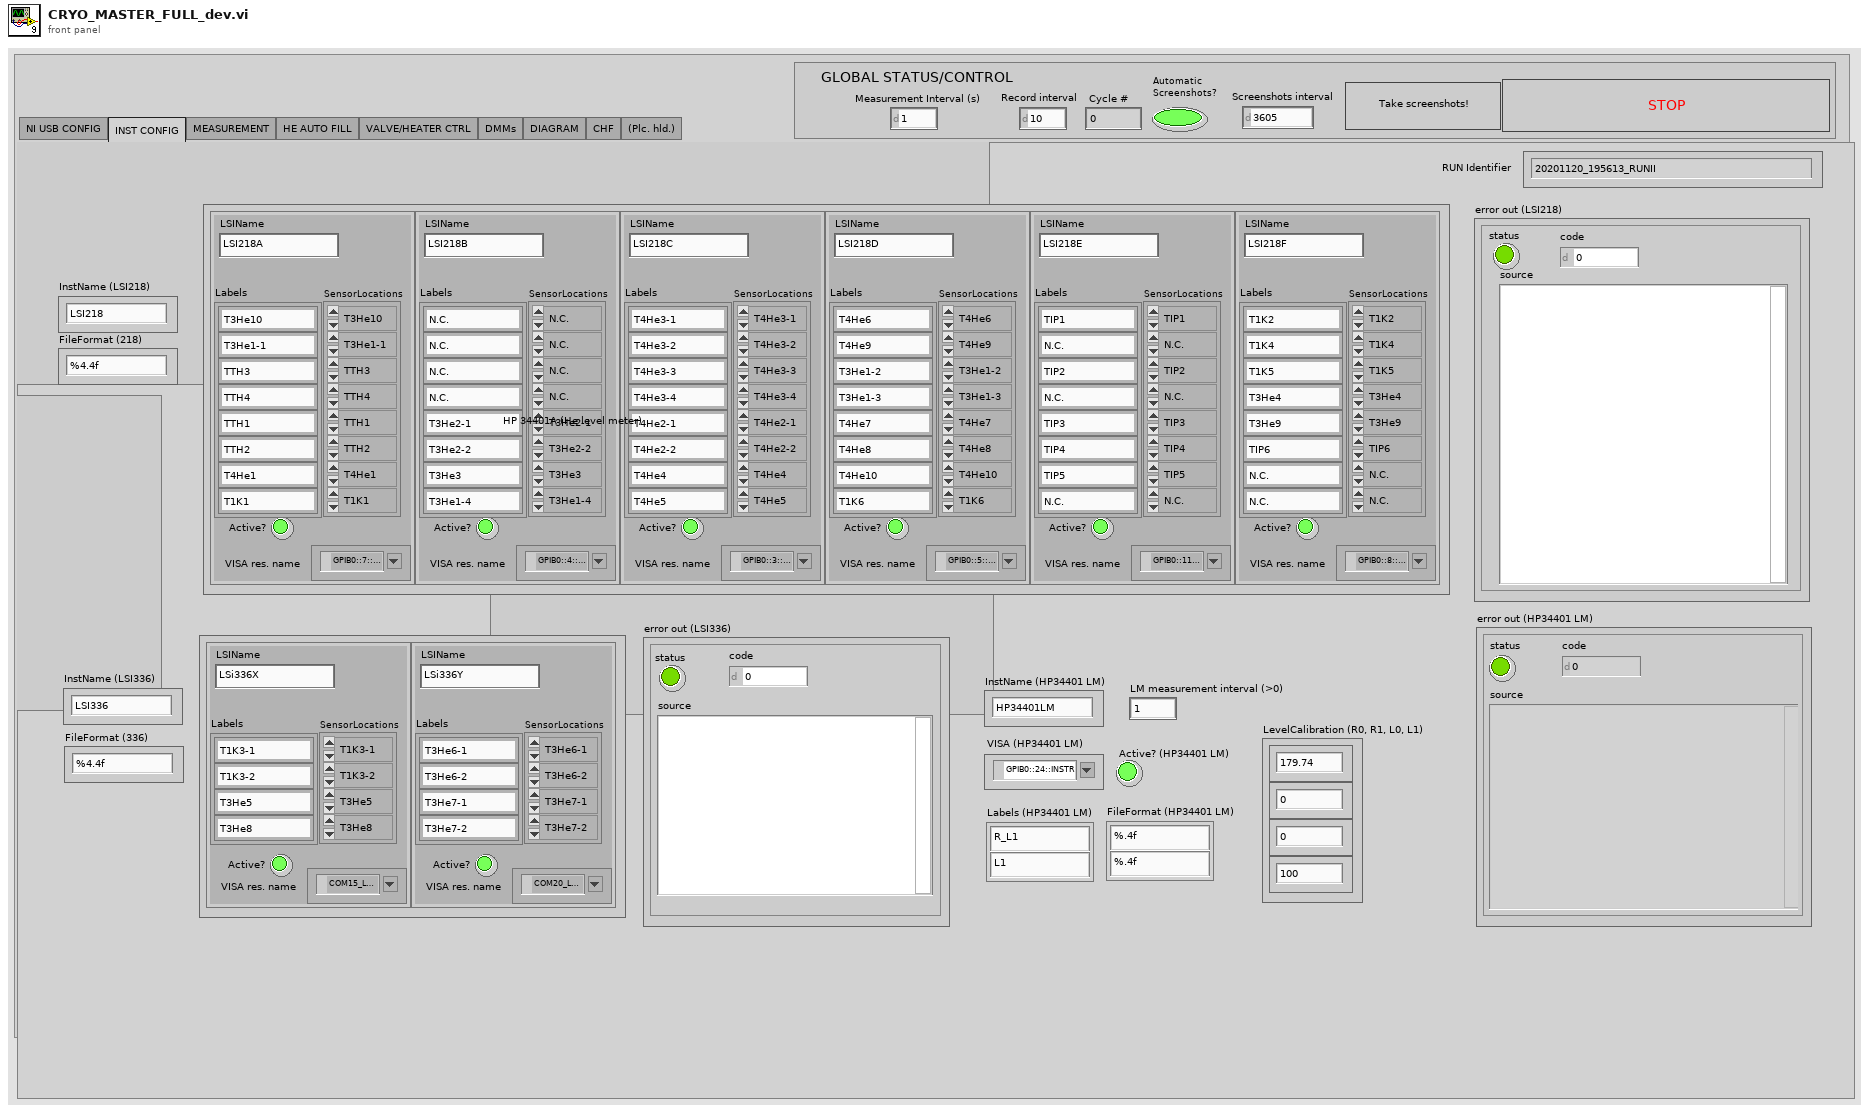
[diagram p1: front panel]
types:
  T1 = enum32{"NI USB CONFIG", "INST CONFIG", "MEASUREMENT", "HE AUTO FILL", "VALVE/HEATER CTRL", "DMMs", "DIAGRAM", "CHF", "(Plc. hld.)"}
  T2 = cluster{"Label":string, "FileFormat":string, "Active?":bool, "Physical CH":tag, " terminal\n type":i32, "ConversionType":cluster{"Type":enum16{"Raw", "SimpleProp", "CC-10_COMBINED", "CC-10_LOG", "LeakDet_EXP", "LeakDet_Mantissa", "Baratron"}, "ConversionParameters":dbl[]}, "VoltageLimits":dbl[]}[]
  T3 = cluster{"LSIName":string, "Labels":string[], "SensorLocations":enum16{"N.C.", "T3He1-1", "T3He1-2", "T3He1-3", "T3He1-4", "T3He2-1", "T3He2-2", "T3He3", "T3He4", "T3He5", "T3He6-1", "T3He6-2", "T3He7-1", "T3He7-2", "T3He8", "T3He9", "T3He10", "T4He1", "T4He2-1", "T4He2-2", "T4He3-1", "T4He3-2", "T4He3-3", "T4He3-4", "T4He4", "T4He5", "T4He6", "T4He7", "T4He8", "T4He9", "T4He10", "T1K1", "T1K2", "T1K3-1", "T1K3-2", "T1K4", "T1K5", "T1K6", "TIP1", "TIP2", "TIP3", "TIP4", "TIP5", "TIP6", "TIP7", "TTH1", "TTH2", "TTH3", "TTH4"}[], "Active?":bool, "VISA res. name":refnum<visa-resource-name>}[]
  T4 = cluster{"TimeArray":timestamp[], "DataArray":dbl[]}[]
  T5 = enum32{"USB6210", "USB6218", "Temeprature (1)", "Temperature (2)", "Temperature (3)"}
  T6 = enum16{"Intialized", "Ready", "Measuring", "Terminated"}
  T7 = enum16{"Initialized", "Ready", "Measuring", "Terminated"}
  T8 = enum16{"USB6210", "USB6218AI", "USB6218AO", "LSI218", "LSI336"}
  T9 = cluster{"TimeArray":timestamp[], "Filtered X":dbl[]}[]
  T10 = cluster{"TimeArray (USB6218)":timestamp[], "DataArrayConv (USB6218)":dbl[]}[]
  T11 = enum16{"USB6210", "USB6218AI", "USB6218AO", "LSI218", "LSI336"}[]
  T12 = cluster{"Label":string, "Active?":bool, "Source":enum16{"USB6210", "USB6218AI", "USB6218AO", "LSI218", "LSI336"}, "SourceLabel":string, "FileFormat":string}[]
  T13 = cluster{"Label":string, "Active?":bool, "VISA resource name":refnum<visa-resource-name>, "Device":enum16{"Agilent34401A", "ADCMT7351", "HP3478A"}, "Measurement":enum16{"DC Volts", "DC Currents", "2-Wire Resistance", "4-Wire Resistance"}, "FileFormat":string}[]
  T14 = enum16{"N.C.", "T3He1-1", "T3He1-2", "T3He1-3", "T3He1-4", "T3He2-1", "T3He2-2", "T3He3", "T3He4", "T3He5", "T3He6-1", "T3He6-2", "T3He7-1", "T3He7-2", "T3He8", "T3He9", "T3He10", "T4He1", "T4He2-1", "T4He2-2", "T4He3-1", "T4He3-2", "T4He3-3", "T4He3-4", "T4He4", "T4He5", "T4He6", "T4He7", "T4He8", "T4He9", "T4He10", "T1K1", "T1K2", "T1K3-1", "T1K3-2", "T1K4", "T1K5", "T1K6", "TIP1", "TIP2", "TIP3", "TIP4", "TIP5", "TIP6", "TIP7", "TTH1", "TTH2", "TTH3", "TTH4"}
  T15 = cluster{"Source":enum16{"USB6210", "USB6218AI", "USB6218AO", "LSI218", "LSI336", "DMMs"}, "SourceLabel":string}
  T16 = cluster{"Source":enum16{"USB6210", "USB6218AI", "USB6218AO", "LSI218", "LSI336", "DMMs"}, "SourceLabel":string, "FileFormat":string}[]
  T17 = cluster{"LSIName":string, "Active?":bool, "LastData":dbl[], "Labels":string[]}[]
  T18 = enum16{"N.C.", "T3He1-1", "T3He1-2", "T3He1-3", "T3He1-4", "T3He2-1", "T3He2-2", "T3He3", "T3He4", "T3He5", "T3He6-1", "T3He6-2", "T3He7-1", "T3He7-2", "T3He8", "T3He9", "T3He10", "T4He1", "T4He2-1", "T4He2-2", "T4He3-1", "T4He3-2", "T4He3-3", "T4He3-4", "T4He4", "T4He5", "T4He6", "T4He7", "T4He8", "T4He9", "T4He10", "T1K1", "T1K2", "T1K3-1", "T1K3-2", "T1K4", "T1K5", "T1K6", "TIP1", "TIP2", "TIP3", "TIP4", "TIP5", "TIP6", "TIP7", "TTH1", "TTH2", "TTH3", "TTH4"}[]
  T19 = cluster{"TimeArray (USB6218)":timestamp[], "DataArrayConv (USB6218)":dbl[]}
  T20 = cluster{"appended array":timestamp[], "ActualCurrentArray":dbl[]}
  T21 = cluster{"appended array":timestamp[], "SetCurrentArray":dbl[]}
  T22 = cluster{"appended array":timestamp[], "SetCurrentArray":dbl[]}[]